vi "GraphsSandbox.vi"() -> ()   [LabVIEW 2016]
uses:
  <vilib>/Utility/miscctls.llb/LVOffsetAndMultiplierTypeDef.ctl
  <vilib>/measure/maresamp.llb/Resample Pair of Arrays (single shot).vi
  <userlib>/_OpenG.lib/array/array.llb/Empty 1D Array (DBL)__ogtk.vi
  <vilib>/measure/NI_MAPro.lvlib
  graph_utilities.lvlib
  <vilib>/Analysis/NI_AALPro.lvlib
panel:
  in  "dt":dbl=1.0 format="%.2p"
  out "XY graphs 2":cluster{dbl[], dbl[]}[](graph)
  out "Numeric":i32
  out "antisymmetric":cluster{dbl[], dbl[]}[](graph)
  out "symmetric":cluster{dbl[], dbl[]}[](graph)
  out "line cuts":cluster{dbl[], dbl[]}[](graph)
  in  "y values to make line cuts":dbl[](array[numeric])=[0.178, 1755.355, 3591.258, 5250.164, 6848.818, 8430.814, 10013.559, 11592.183, 13170.614, 14750.752, 16322.644, 17884.434, 19454.629, 21018.842, 22584.172, 24140.527, 25702.117, 27263.146, 28814.635, 30370.051, 31928.646, 33482.563, 35026.938, 36578.797, 38130.281, 39680.648, 41220.531, 42767.34, 44311.715, 45856.09, 47392.793, 48933.426, 50466.949, 52013.754, 53544.66, 55082.859, 56617.504, 58146.348, 59678.0, 61211.707, 62741.488, 64267.715, 65796.563, 67326.156, 68845.461, 70371.867, 71899.031, 73423.758, 74939.883, 76462.93, 77982.977, 79499.102, 81016.906, 82537.516, 84054.578, 85563.961, 87080.086, 88593.969, 89996.516] format="%#_6p"
  out "resampled intensity graph":dbl[][](graph)
  in  "XY graphs":cluster{dbl[], dbl[]}[](graph)
  in  "\"y\" array (each curve's parameter)":dbl[](array[numeric])=[0.178, 1755.355, 3591.258, 5250.164, 6848.818, 8430.814, 10013.559, 11592.183, 13170.614, 14750.752, 16322.644, 17884.434, 19454.629, 21018.842, 22584.172, 24140.527, 25702.117, 27263.146, 28814.635, 30370.051, 31928.646, 33482.563, 35026.938, 36578.797, 38130.281, 39680.648, 41220.531, 42767.34, 44311.715, 45856.09, 47392.793, 48933.426, 50466.949, 52013.754, 53544.66, 55082.859, 56617.504, 58146.348, 59678.0, 61211.707, 62741.488, 64267.715, 65796.563, 67326.156, 68845.461, 70371.867, 71899.031, 73423.758, 74939.883, 76462.93, 77982.977, 79499.102, 81016.906, 82537.516, 84054.578, 85563.961, 87080.086, 88593.969, 89996.516] format="%#_6p"
  # "1. convert x and y arrays to x and y scales for intensity graph"
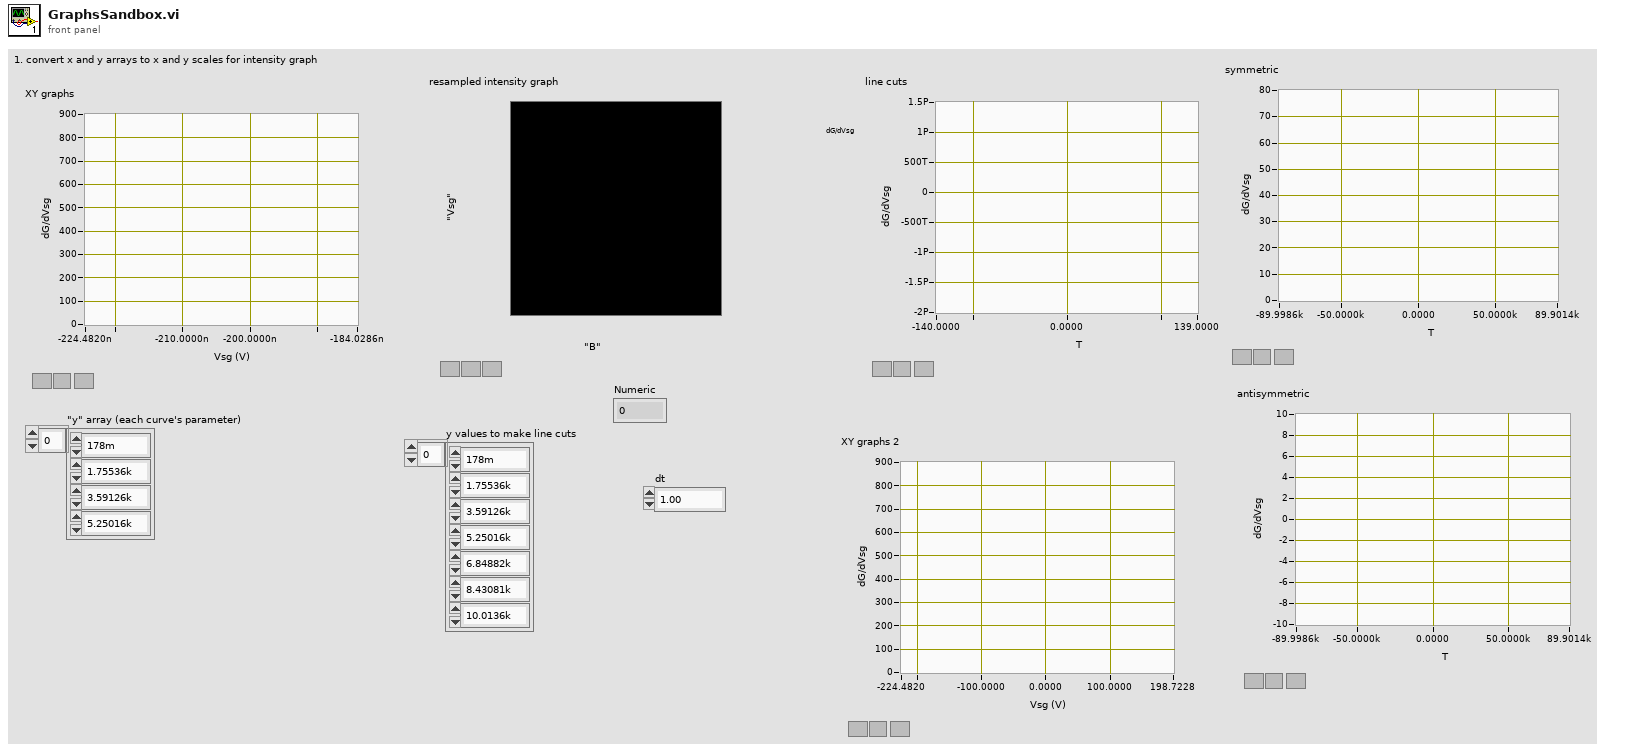
[diagram p1: front panel]
types:
  T1 = cluster{"x array":dbl[], "\"y\" array (parms)":dbl[], "XY graphs":cluster{dbl[], dbl[]}[]}
  T2 = cluster{"Decimated Array":dbl[], "Decimated Array":dbl[]}
  T3 = typedef "LVOffsetAndMultiplierTypeDef.ctl" = cluster{"Offset":dbl, "Multiplier":dbl}
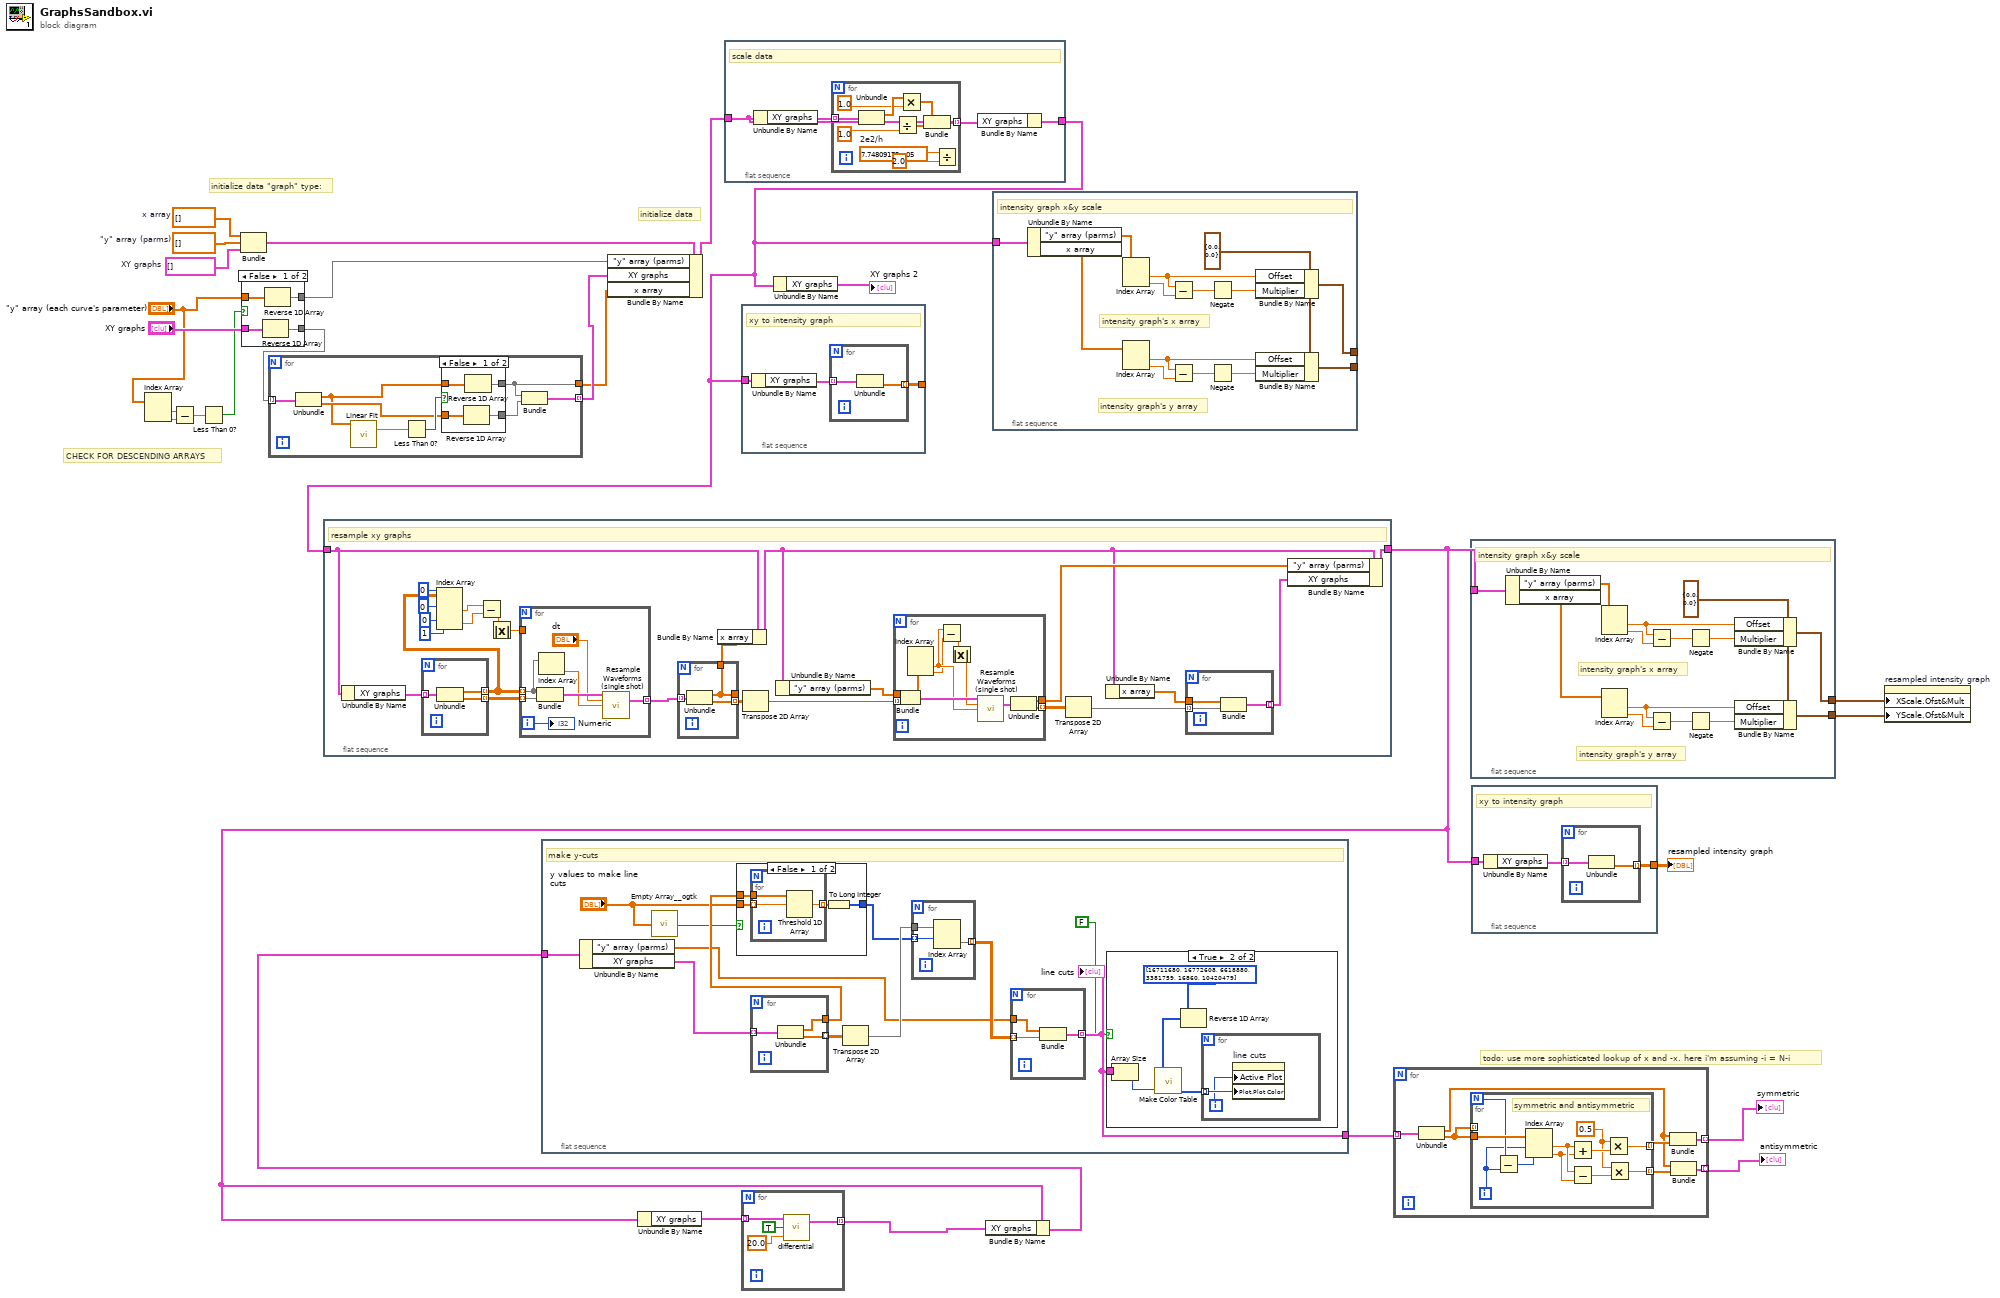
[diagram p0: block diagram]
diagram:
  w26 = dbl[] []  # x array
  w25 = cluster{dbl[], dbl[]}[] []  # XY graphs
  w27 = dbl[] []  # "y" array (parms)
  # "initialize data \"graph\" type:"
  # "todo: use more sophisticated lookup of x and -x. here i'm assuming -i = N-i"
  # "CHECK FOR DESCENDING ARRAYS"
  # "initialize data"
  n1 = Index Array(array="\"y\" array (each curve's parameter)") -> (element #1=w9:dbl, element #2=w10:dbl)  [unwired: 2 in]
  n2 = Subtract(x=w9, y=w10) -> (x-y=w8:dbl)
  n3 = Less Than 0?(x=w8) -> (x < 0?=w7:bool)
  n4 = Bundle("x array"=w26, "\"y\" array (parms)"=w27, "XY graphs"=w25) -> (w24:T1)  [unwired: 1 in]
  n5 = case shown="False" w7 {
    tunnel: "XY graphs" -> [w31 w32]
    tunnel: [w30 w32] -> w5
    tunnel: [w29 w33] -> w12
    tunnel: "\"y\" array (each curve's parameter)" -> [w28 w33]
    frame False {
      n6 = Reverse 1D Array(array=w31) -> (reversed array=w30:cluster{dbl[], dbl[]}[])
      n7 = Reverse 1D Array(array=w28) -> (reversed array=w29:dbl[])
    }
    frame True {
    }
  }
  n8 = for {
    tunnel: w5 -> [w41] mode=indexing
    tunnel: [w37] -> w4 mode=indexing
    tunnel: [w36] -> w3
    n9 = Unbundle(w41) -> (w35:dbl[], w39:dbl[])
    n10 = call <vilib>:"Linear Fit.vi"("Y"=w35) -> ("slope"=w34:dbl)  [unwired: 10 in, 4 out]
    n11 = Less Than 0?(x=w34) -> (x < 0?=w40:bool)
    n12 = case shown="False" w40 {
      tunnel: w39 -> [w45 w46]
      tunnel: [w44 w46] -> w38
      tunnel: [w43 w47] -> w36
      tunnel: w35 -> [w42 w47]
      frame False {
        n13 = Reverse 1D Array(array=w45) -> (reversed array=w44:dbl[])
        n14 = Reverse 1D Array(array=w42) -> (reversed array=w43:dbl[])
      }
      frame True {
      }
    }
    n15 = Bundle(w36, w38) -> (w37:cluster{dbl[], dbl[]})  [unwired: 1 in]
  }
  n16 = flat-sequence {
    tunnel: [w63] -> w6
    tunnel: w2 -> [w50]
    frame #0 {
      # "resample xy graphs"
      n17 = Unbundle By Name(w50) -> ("XY graphs"=w62:cluster{dbl[], dbl[]}[])
      n18 = for {
        tunnel: w62 -> [w74] mode=indexing
        tunnel: [w73] -> w61 mode=indexing
        tunnel: [w72] -> w56 mode=indexing
        n19 = Unbundle(w74) -> (w72:dbl[], w73:dbl[])
      }
      n20 = Index Array(array=w56, index (row) #1=0 ("index (row)"), index (col) #1=0 ("disabled index (col)"), index (row) #2=0 ("index (row)"), index (col) #2=1 ("disabled index (col)")) -> (element #1=w59:dbl, element #2=w57:dbl)
      n21 = Subtract(x=w59, y=w57) -> (x-y=w58:dbl)
      n22 = Absolute Value(x=w58) -> (abs(x)=w55:dbl)
      n23 = for {
        tunnel: w56 -> [w76] mode=indexing
        tunnel: w61 -> [w80] mode=indexing
        tunnel: [w79] -> w60 mode=indexing
        tunnel: w55 -> [_]
        i -> [w78]
        n24 = Bundle(w76, w80) -> (w81:cluster{dbl[], dbl[]})  [unwired: 1 in]
        n25 = Index Array(array=w76) -> (element=w75:dbl)  [unwired: 1 in]
        n26 = call-poly <vilib>:"Resample Waveforms (single shot).vi"("XY-data in"=w81, "dt"="dt", "t0"=w75) -> ("XY-data out"=w79:cluster{"X-array":dbl[], "Y-array":dbl[]})  [unwired: 8 in, 4 out]
        "Numeric" <- w78
      }
      n27 = for {
        tunnel: w60 -> [w84] mode=indexing
        tunnel: [w83] -> w68 mode=indexing
        tunnel: [w82] -> _
        tunnel: [w82] -> w49
        n28 = Unbundle(w84) -> ("X-array"=w82:dbl[], "Y-array"=w83:dbl[])
      }
      n29 = Bundle By Name(cluster=w50, "x array"=w49) -> (w48:T1)
      n30 = Transpose 2D Array(2D array=w68) -> (transposed array=w71:dbl[][])
      n31 = Unbundle By Name(w48) -> ("\"y\" array (parms)"=w67:dbl[])
      n32 = for {
        tunnel: w71 -> [w97] mode=indexing
        tunnel: w67 -> [w95]
        tunnel: [w92] -> w70 mode=indexing
        tunnel: [w91] -> w65
        n33 = Bundle("\"y\" array (parms)"=w95, w97) -> (w96:cluster{"\"y\" array (parms)":dbl[], dbl[]})  [unwired: 1 in]
        n34 = Index Array(array=w95) -> (element #1=w94:dbl, element #2=w93:dbl)  [unwired: 2 in]
        n35 = Subtract(x=w94, y=w93) -> (x-y=w89:dbl)
        n36 = Absolute Value(x=w89) -> (abs(x)=w88:dbl)
        n37 = call-poly <vilib>:"Resample Waveforms (single shot).vi"("XY-data in"=w96, "dt"=w88, "t0"=w94) -> ("XY-data out"=w90:cluster{"X-array":dbl[], "Y-array":dbl[]})  [unwired: 8 in, 4 out]
        n38 = Unbundle(w90) -> ("X-array"=w91:dbl[], "Y-array"=w92:dbl[])
      }
      n39 = Transpose 2D Array(2D array=w70) -> (transposed array=w69:dbl[][])
      n40 = Unbundle By Name(w48) -> ("x array"=w66:dbl[])
      n41 = for {
        tunnel: w69 -> [w87] mode=indexing
        tunnel: w66 -> [w86]
        tunnel: [w85] -> w64 mode=indexing
        n42 = Bundle("x array"=w86, w87) -> (w85:cluster{"x array":dbl[], dbl[]})  [unwired: 1 in]
      }
      n43 = Bundle By Name(cluster=w48, "\"y\" array (parms)"=w65, "XY graphs"=w64) -> (w63:T1)
    }
  }
  n44 = flat-sequence {
    tunnel: [w100] -> w18
    tunnel: w14 -> [w99]
    frame #0 {
      # "make y-cuts"
      n45 = Unbundle By Name(w99) -> ("\"y\" array (parms)"=w103:dbl[], "XY graphs"=w109:cluster{dbl[], dbl[]}[])
      n46 = call-poly <userlib>:"Empty Array__ogtk.vi"("Array"="y values to make line cuts") -> ("Empty Array?"=w101:bool)  [unwired: 8 in]
      n47 = for {
        tunnel: w109 -> [w135] mode=indexing
        tunnel: [w134] -> w108 mode=indexing
        tunnel: [w133] -> w104
        n48 = Unbundle(w135) -> (w133:dbl[], w134:dbl[])
      }
      n49 = case shown="False" w101 {
        tunnel: [w117 w124] -> w106
        tunnel: w104 -> [w119 w125]
        tunnel: "y values to make line cuts" -> [w118 _]
        frame False {
          n50 = for {
            tunnel: w119 -> [w123]
            tunnel: w118 -> [w122] mode=indexing
            tunnel: [w121] -> w120 mode=indexing
            n51 = Threshold 1D Array(2:w122, 3:w123) -> (0:w121:dbl)  [unwired: 1 in]
          }
          n52 = To Long Integer(number=w120) -> (32bit integer=w117:i32[])
        }
        frame True {
          n53 = for {
            tunnel: w125 -> [_] mode=indexing
            tunnel: [w126] -> w124 mode=indexing
            i -> [w126]
          }
        }
      }
      n54 = Transpose 2D Array(2D array=w108) -> (transposed array=w107:dbl[][])
      n55 = for {
        tunnel: w107 -> [w132]
        tunnel: w106 -> [w131] mode=indexing
        tunnel: [w130] -> w105 mode=indexing
        n56 = Index Array(array=w132, index (row)=w131) -> (element=w130:dbl[])  [unwired: 1 in]
      }
      n57 = for {
        tunnel: w105 -> [w129] mode=indexing
        tunnel: w103 -> [w128]
        tunnel: [w127] -> w100 mode=indexing
        n58 = Bundle("\"y\" array (parms)"=w128, w129) -> (w127:cluster{"\"y\" array (parms)":dbl[], dbl[]})  [unwired: 1 in]
      }
      "line cuts" <- w100
      n59 = case shown="True" FALSE {
        tunnel: w100 -> [_ w110]
        frame False {
        }
        frame True {
          n60 = Array Size(array=w110) -> (size(s)=w114:i32)
          n61 = Reverse 1D Array(array=u32[] [16711680, 16772608, 6618880, 3381759, 16860, 10420479] ("color scale")) -> (reversed array=w111:u32[])
          n62 = call "Make Color Table.vi"("Colors []"=w111, "Size"=w114) -> ("Color Tbl"=w112:u32[])  [unwired: 3 out]
          n63 = for {
            tunnel: w112 -> [w116] mode=indexing
            i -> [w115]
            n64 = property on="line cuts" class="XYGraph (strict)"("Active Plot"=w115, "Plot.Plot Color"=w116) -> ()  [unwired: 2 in, 2 out]
          }
        }
      }
    }
  }
  n65 = Bundle By Name(cluster=w24, "\"y\" array (parms)"=w12, "XY graphs"=w4, "x array"=w3) -> (w15:T1)
  n66 = Unbundle By Name(w6) -> ("XY graphs"=w20:cluster{dbl[], dbl[]}[])
  n67 = flat-sequence {
    tunnel: w15 -> [w137]
    tunnel: [w136] -> w2
    frame #0 {
      # "scale data"
      n68 = Unbundle By Name(w137) -> ("XY graphs"=w139:cluster{dbl[], dbl[]}[])
      n69 = for {
        tunnel: w139 -> [w149] mode=indexing
        tunnel: [w144] -> w138 mode=indexing
        w143 = 7.74809173e-05  # 2e2/h
        n70 = Unbundle(w149) -> (w146:dbl[], w148:dbl[])
        n71 = Divide(x=w148, y=1.0) -> (x/y=w147:dbl[])
        n72 = Multiply(x=w146, y=1.0) -> (x*y=w141:dbl[])
        n73 = Bundle(w141, w147) -> (w144:cluster{dbl[], dbl[]})  [unwired: 1 in]
        n74 = Divide(x=w143, y=2.0) -> ()  [unwired: 1 out]
      }
      n75 = Bundle By Name(cluster=w137, "XY graphs"=w138) -> (w136:T1)
    }
  }
  n76 = flat-sequence {
    tunnel: w2 -> [w151]
    tunnel: [w150] -> _
    frame #0 {
      # "xy to intensity graph"
      n77 = Unbundle By Name(w151) -> ("XY graphs"=w152:cluster{dbl[], dbl[]}[])
      n78 = for {
        tunnel: w152 -> [w154] mode=indexing
        tunnel: [w153] -> w150 mode=indexing
        n79 = Unbundle(w154) -> (w153:dbl[])  [unwired: 1 out]
      }
    }
  }
  n80 = for {
    tunnel: w20 -> [w158] mode=indexing
    tunnel: [w155] -> w19 mode=indexing
    n81 = call <userlib>:"differential.vi"("Numeric"=20.0, "dy/dx vs x"=TRUE, "A vs B 2"=w158) -> ("A vs B 3"=w155:T2)  [unwired: 1 in]
  }
  n82 = Unbundle By Name(w2) -> ("XY graphs"=→"XY graphs 2":cluster{dbl[], dbl[]}[])
  n83 = Bundle By Name(cluster=w6, "XY graphs"=w19) -> (w14:T1)
  n84 = flat-sequence {
    tunnel: [w172] -> _
    tunnel: [w162] -> _
    tunnel: w2 -> [w159]
    frame #0 {
      w163 = T3 {"Offset"=0.0, "Multiplier"=0.0} ("X Scale.Offset and Multiplier")
      # "intensity graph's y array"
      # "intensity graph's x array"
      # "intensity graph x&y scale"
      n85 = Unbundle By Name(w159) -> ("\"y\" array (parms)"=w161:dbl[], "x array"=w160:dbl[])
      n86 = Index Array(array=w161) -> (element #1=w166:dbl, element #2=w171:dbl)  [unwired: 2 in]
      n87 = Index Array(array=w160) -> (element #1=w164:dbl, element #2=w168:dbl)  [unwired: 2 in]
      n88 = Subtract(x=w166, y=w171) -> (x-y=w170:dbl)
      n89 = Subtract(x=w164, y=w168) -> (x-y=w169:dbl)
      n90 = Negate(x=w170) -> (-x=w167:dbl)
      n91 = Negate(x=w169) -> (-x=w165:dbl)
      n92 = Bundle By Name(cluster=w163, "Offset"=w166, "Multiplier"=w167) -> (w172:T3)
      n93 = Bundle By Name(cluster=w163, "Offset"=w164, "Multiplier"=w165) -> (w162:T3)
    }
  }
  n94 = for {
    tunnel: w18 -> [w179] mode=indexing
    tunnel: [w174] -> w17 mode=indexing
    tunnel: [w173] -> w16 mode=indexing
    n95 = Unbundle(w179) -> ("\"y\" array (parms)"=w175:dbl[], w178:dbl[])
    n96 = for {
      N -> [w189]
      tunnel: w178 -> [w190]
      tunnel: w178 -> [_] mode=indexing
      tunnel: [w181] -> w177 mode=indexing
      tunnel: [w180] -> w176 mode=indexing
      i -> [w188]
      w182 = 0.5 ("x")
      # "symmetric and antisymmetric"
      n97 = Subtract(x=w189, y=w188) -> (x-y=w187:i32)
      n98 = Index Array(array=w190, index #1=w188, index #2=w187) -> (element #1=w186:dbl, element #2=w185:dbl)
      n99 = Add(x=w186, y=w185) -> (x+y=w184:dbl)
      n100 = Subtract(x=w186, y=w185) -> (x-y=w183:dbl)
      n101 = Multiply(x=w182, y=w184) -> (x*y=w181:dbl)
      n102 = Multiply(x=w182, y=w183) -> (x*y=w180:dbl)
    }
    n103 = Bundle("\"y\" array (parms)"=w175, w177) -> (w174:cluster{"\"y\" array (parms)":dbl[], dbl[]})  [unwired: 1 in]
    n104 = Bundle("\"y\" array (parms)"=w175, w176) -> (w173:cluster{"\"y\" array (parms)":dbl[], dbl[]})  [unwired: 1 in]
  }
  "antisymmetric" <- w16
  "symmetric" <- w17
  n105 = flat-sequence {
    tunnel: [w204] -> w22
    tunnel: [w194] -> w21
    tunnel: w6 -> [w191]
    frame #0 {
      w195 = T3 {"Offset"=0.0, "Multiplier"=0.0} ("X Scale.Offset and Multiplier")
      # "intensity graph's y array"
      # "intensity graph's x array"
      # "intensity graph x&y scale"
      n106 = Unbundle By Name(w191) -> ("\"y\" array (parms)"=w193:dbl[], "x array"=w192:dbl[])
      n107 = Index Array(array=w193) -> (element #1=w198:dbl, element #2=w203:dbl)  [unwired: 2 in]
      n108 = Index Array(array=w192) -> (element #1=w196:dbl, element #2=w200:dbl)  [unwired: 2 in]
      n109 = Subtract(x=w198, y=w203) -> (x-y=w202:dbl)
      n110 = Subtract(x=w196, y=w200) -> (x-y=w201:dbl)
      n111 = Negate(x=w202) -> (-x=w199:dbl)
      n112 = Negate(x=w201) -> (-x=w197:dbl)
      n113 = Bundle By Name(cluster=w195, "Offset"=w198, "Multiplier"=w199) -> (w204:T3)
      n114 = Bundle By Name(cluster=w195, "Offset"=w196, "Multiplier"=w197) -> (w194:T3)
    }
  }
  n115 = flat-sequence {
    tunnel: [w206] -> w23
    tunnel: w6 -> [w205]
    frame #0 {
      # "xy to intensity graph"
      n116 = Unbundle By Name(w205) -> ("XY graphs"=w207:cluster{dbl[], dbl[]}[])
      n117 = for {
        tunnel: w207 -> [w209] mode=indexing
        tunnel: [w208] -> w206 mode=indexing
        n118 = Unbundle(w209) -> (w208:dbl[])  [unwired: 1 out]
      }
    }
  }
  n119 = property on="resampled intensity graph" class="IntGraph (strict)"("XScale.Ofst&Mult"=w22, "YScale.Ofst&Mult"=w21) -> ()  [unwired: 2 in, 2 out]
  "resampled intensity graph" <- w23
